vi "SMain.vi"() -> ()   [LabVIEW 2011] (continued)
                            n1009 = Build Path(base path=w1648, name or relative path="TXT\\ReportInf.txt" ("名称或相对路径")) -> (appended path=w1644:path)
                            n1010 = Write to Text File(file (use dialog)=w1644, text=w1645) -> ()  [unwired: 2 in, 3 out]
                          }
                          frame #14 {
                            # "生成报告"
                            n1011 = property on="MO:" class="Str"() -> ("Visible"=w1720:bool)  [unwired: 2 in, 2 out]
                            n1012 = case shown="真" w1720 {
                              tunnel: w1727 -> [_ w1752]
                              frame False {
                              }
                              frame True {
                                w1732 = "0"
                                w1733 = "1"
                                n1013 = property class="Str"(reference=w1752) -> (reference out=w1745:refnum<vi>, "Value"=w1746:string)  [unwired: 1 in, 1 out]
                                n1014 = local read "DB1"() -> (w1728:T8)
                                n1015 = local read "test result"() -> (w1743:bool)
                                n1016 = local read "MO:"() -> (w1750:string)
                                n1017 = local read "P/N:"() -> (w1751:string)
                                n1018 = call "按工单数量查询.vi"("MO"=w1750, "DBSet"=w1728, "test result"=w1743, "PN"=w1751) -> ("当前数量"=w1742:string)  [unwired: 5 in]
                                n1019 = Decimal String To Number(string=w1742) -> (number=w1741:i32)  [unwired: 2 in, 1 out]
                                n1020 = local write "Pro Num"(w1741) -> ()
                                n1021 = Concatenate Strings(w1746, "\n", "当前工单已生产：" ("字符串"), w1742, "条" ("字符串")) -> (w1744:string)
                                n1022 = local read "MO Num"() -> (w1739:i64)
                                n1023 = local read "Pro Num"() -> (w1740:i64)
                                n1024 = property class="Str"(reference=w1745, "Value"=w1744) -> ()  [unwired: 1 in, 2 out]
                                n1025 = Subtract(x=w1740, y=w1739) -> (x-y=w1737:i64)
                                n1026 = Greater?(x=w1737, y=i64 0) -> (0:w1735:bool)
                                n1027 = Greater?(x=w1737, y=i64 20) -> (0:w1734:bool)
                                n1028 = Select(t=w1733, s=w1735, f=w1732) -> (s? t:f=w1731:string)
                                n1029 = Select(t=w1733, s=w1734, f=w1732) -> (s? t:f=w1730:string)
                                n1030 = Concatenate Strings(w1731, w1730) -> (w1729:string)
                                n1031 = case shown="\"10\"" w1729 {
                                frame "00", Default {
                                w1753 = u32 0
                                n1032 = property on="Pro Num" class="DigNum (严格)"("NumText.TextColor"=w1753) -> ()  [unwired: 2 in, 2 out]
                                n1033 = property on="P/N:" class="Str"("Text.TextColor"=w1753) -> ()  [unwired: 2 in, 2 out]
                                }
                                frame "10" {
                                w1754 = u32 16772608
                                n1034 = property on="Pro Num" class="DigNum (严格)"("NumText.TextColor"=w1754) -> ()  [unwired: 2 in, 2 out]
                                n1035 = property on="P/N:" class="Str"("Text.TextColor"=w1754) -> ()  [unwired: 2 in, 2 out]
                                }
                                frame "11" {
                                w1755 = u32 14423296
                                n1036 = property on="Pro Num" class="DigNum (严格)"("NumText.TextColor"=w1755) -> ()  [unwired: 2 in, 2 out]
                                n1037 = property on="P/N:" class="Str"("Text.TextColor"=w1755) -> ()  [unwired: 2 in, 2 out]
                                }
                                }
                              }
                            }
                            n1038 = local read "Report Temp. Name"() -> (w1725:string)
                            n1039 = local read "TXT Data Path"() -> (w1719:path)
                            n1040 = local read "Report Config"() -> (w1724:string[])
                            n1041 = local read "Report Inf"() -> (w1723:string[])
                            n1042 = local read "Excel?"() -> (w1726:bool)
                            n1043 = Strip Path(path=w1719) -> (stripped path=w1718:path)  [unwired: 1 out]
                            n1044 = case shown="真" w1726 {
                              tunnel: w1719 -> [_ w1757]
                              tunnel: w1725 -> [_ w1768]
                              tunnel: w1724 -> [_ w1769]
                              tunnel: w1723 -> [_ w1764]
                              tunnel: w1722 -> [_ w1758]
                              tunnel: w1718 -> [_ w1756]
                              frame False {
                              }
                              frame True {
                                n1045 = Index Array(array=w1769, index #1=0 ("索引")) -> (element #1=w1765:string, element #2=w1763:string)  [unwired: 1 in]
                                n1046 = String To Path(string=w1768) -> (path=w1767:path)
                                n1047 = call "Excel Config.vi"("Config String"=w1765) -> ("Start(0,0)"=w1772:cluster{i32, i32}[], "Sheet Number List"=w1771:i32[], "File Name List"=w1770:string[])  [unwired: 8 in]
                                n1048 = call "Excel Config.vi"("Config String"=w1763) -> ("Start(0,0)"=w1762:cluster{i32, i32}[])  [unwired: 8 in, 2 out]
                                n1049 = call "Excel Export.vi"("template Path"=w1767, "Data Basic Path"=w1757, "File Name List"=w1770, "Sheet Index List"=w1771, "Report Inf"=w1764, "Inf start"=w1762, "Sheet start(0,0)"=w1772, "Demo"=w1758, "Report Type"="Report Type:", "reportSavePath"=w1756, "StartPage"="Start Page", "EndPage"="End Page") -> ()  [unwired: 15 in, 1 out]
                              }
                            }
                            n1050 = local write "proBar"(u8 90 ("proBar")) -> ()
                          }
                          frame #15 {
                            (unwired) FALSE
                            # "上传测试数据"
                            n1051 = local read "EEPROMTF"() -> (w1777:bool)
                            n1052 = local read "upload"() -> (w1776:bool)
                            n1053 = local read "测试模式"() -> (w1775:bool)
                            n1054 = Or(x=w1776, y=w1777) -> (x .or. y?=w1774:bool)
                            n1055 = And(x=w1774, y=w1775) -> (x .and. y?=w1773:bool)
                            n1056 = case shown="真" w1773 {
                              tunnel: w1778 -> [_ w1780]
                              frame False {
                                n1057 = local write "proBar"(u8 99 ("proBar")) -> ()
                              }
                              frame True {
                                n1058 = case shown="假" w1780 {
                                frame True {
                                n1059 = local read "strFSN 原始SN"() -> (w1785:string)
                                n1060 = local read "NetPathCompress1"() -> (w1783:path)
                                n1061 = local read "NetCmdCompress"() -> (w1784:string)
                                n1062 = local read "NetPathCompress2"() -> (w1782:path)
                                n1063 = call <vilib>:"Application Directory.vi"() -> ("Application Directory"=w1788:path)
                                n1064 = Build Path(base path=w1788, name or relative path="Demo_data") -> (appended path=w1786:path)
                                n1065 = local read "EEPROMTF"() -> (w1793:bool)
                                n1066 = local read "db_VNA"() -> (w1791:string)
                                n1067 = local read "条码输出"() -> (w1789:string)
                                n1068 = local read "Excel?"() -> (w1792:bool)
                                n1069 = local read "P/N:"() -> (w1794:string)
                                n1070 = local read "S/N:"() -> (w1790:string)
                                n1071 = call "compressFiles-Demo.vi"("mis原始sn字符串"=w1785, "P/N:"=w1794, "NetPathCompress1"=w1783, "NetPathCompress2"=w1782, "NetCmdCompress"=w1784, "original Path"=w1786, "EEPROMTF"=w1793, "Excel?"=w1792, "db_VNA"=w1791, "S/N:"=w1790, "条码输出"=w1789) -> ()  [unwired: 5 in]
                                }
                                frame False {
                                n1072 = local read "重测原因"() -> (w1797:string)
                                n1073 = property on="测试模式" class="Ring (严格)"() -> ("RingText.Text"=w1796:string)  [unwired: 2 in, 2 out]
                                n1074 = property on="线别" class="Ring (严格)"() -> ("RingText.Text"=w1795:string)  [unwired: 2 in, 2 out]
                                n1075 = local read "MO:"() -> (w1798:string)
                                n1076 = local read "Current Testing Label/当前测试条码"() -> (w1809:string)
                                n1077 = local read "要烧录的时间和Sn"() -> (w1802:string)
                                n1078 = local read "NetCmdCompress"() -> (w1799:string)
                                n1079 = local read "NetPathCompress1"() -> (w1800:path)
                                n1080 = local read "customer date"() -> (w1808:string)
                                n1081 = local read "strFSN 原始SN"() -> (w1811:string)
                                n1082 = local read "NetPathCompress2"() -> (w1801:path)
                                n1083 = local read "未经进制转换的sn(客户 jin zhi sn)"() -> (w1803:string)
                                n1084 = local read "Shi jin zhi sn"() -> (w1807:string)
                                n1085 = local read "midVar_time_date"() -> (w1806:timestamp)
                                n1086 = Format Date/Time String(time format string (%c)="%Y%m%d" ("时间格式字符串(%c)"), seconds (now)=w1806) -> (date/time string=w1804:string)  [unwired: 1 in]
                                n1087 = local read "original Path"() -> (w1812:path)
                                n1088 = local read "EEPROMTF"() -> (w1817:bool)
                                n1089 = local read "db_VNA"() -> (w1815:string)
                                n1090 = local read "条码输出"() -> (w1813:string)
                                n1091 = local read "Excel?"() -> (w1816:bool)
                                n1092 = local read "P/N:"() -> (w1818:string)
                                n1093 = local read "S/N:"() -> (w1814:string)
                                n1094 = local read "要烧录的DateCode"() -> (w1810:string)
                                n1095 = call "compressFiles.vi"("original Path"=w1812, "重测原因"=w1797, "NetPathCompress2"=w1801, "EEPROMTF"=w1817, "Excel?"=w1816, "测试模式"=w1796, "db_VNA"=w1815, "P/N:"=w1818, "S/N:"=w1814, "测试线别"=w1795, "NetPathCompress1"=w1800, "NetCmdCompress"=w1799, "mis原始sn字符串"=w1811, "条码输出"=w1813, "eprm_datecode"=w1810, "eprm_dateAndsn"=w1802, "itsn_really"=w1809, "label_date"=w1808, "decimel_sn"=w1807, "label_sn"=w1803, "decimel_date"=w1804, "MO"=w1798) -> ()  [unwired: 6 in]
                                }
                                }
                                n1096 = local write "proBar"(u8 95 ("proBar")) -> ()
                              }
                            }
                          }
                          frame #16 {
                            n1097 = flat-sequence {
                              frame #0 {
                                n1098 = local read "AutoSN"() -> (w1819:bool)
                                n1099 = call "运行批处理.vi"() -> ()  [unwired: 12 in]
                                n1100 = local write "proBar"(u8 100 ("proBar")) -> ()
                                n1101 = case shown="假" w1819 {
                                frame False {
                                n1102 = local write "S/N:"("" ("S/N:")) -> ()
                                n1103 = property on="S/N:" class="Str"("DisabledEnum"=T17."Enabled" ("禁用")) -> ()  [unwired: 2 in, 2 out]
                                }
                                frame True {
                                n1104 = local write "S/N:"("automatic sn" ("S/N:")) -> ()
                                n1105 = property on="S/N:" class="Str"("DisabledEnum"=T17."Disabled and Grayed Out" ("禁用")) -> ()  [unwired: 2 in, 2 out]
                                }
                                }
                                n1106 = disable-structure shown="启用" {
                                frame Disabled {
                                n1107 = call <vilib>:"System Exec.vi"("run minimized? (F)"=TRUE, "command line"="taskkill /IM bartend.exe /F") -> ()  [unwired: 6 in, 4 out]
                                }
                                frame Enabled {
                                }
                                }
                              }
                              frame #1 {
                                w1827 = FALSE ("Urgent Stop")
                                w1831 = 0
                                n1108 = property on="Start Test" class="Bool"("DisabledEnum"=w1831) -> ()  [unwired: 2 in, 2 out]
                                n1109 = property on="Tab_Graph" class="TabCtl (严格)"("Value"=w1831) -> ()  [unwired: 2 in, 2 out]
                                n1110 = property on="Urgent Stop" class="Bool (严格)"("DisabledEnum"=2 ("索引")) -> ()  [unwired: 2 in, 2 out]
                                n1111 = local write "State"("wait" ("state")) -> ()
                                n1112 = local write "Urgent Stop"(w1827) -> ()
                                n1113 = global write "全局.vi" "manual stop"(w1827) -> ()
                                n1114 = property on="S/N:" class="Str"("Key Focus"=TRUE ("键选中")) -> ()  [unwired: 2 in, 2 out]
                              }
                            }
                          }
                        }
                      }
                    }
                  }
                }
              }
              frame #3 {
                n1115 = local read "caliFlag"() -> (w1832:string)
                n1116 = case shown="\"假\", 默认" w1832 {
                  frame "假", Default {
                  }
                  frame "cali" {
                    n1117 = local write "State"("datacheck" ("state")) -> ()
                    n1118 = property on="Start Test" class="Bool"("DisabledEnum"=T17."Disabled and Grayed Out" ("禁用")) -> ()  [unwired: 2 in, 2 out]
                    n1119 = property on="Tab_Graph" class="TabCtl (严格)"("Value"=T15."Sxxxx1" ("Tab_Graph")) -> ()  [unwired: 2 in, 2 out]
                  }
                }
              }
            }
          }
          frame "datacheck" {
            n1120 = stacked-sequence {
              frame #0 {
                n1121 = local read "original Path"() -> (w1841:path)
                n1122 = Build Path(base path=w1841, name or relative path="txt" ("名称或相对路径")) -> (appended path=w1836:path)
                n1123 = call "caliCalcu.vi"("basic"=w1836) -> ("FileExsit"=w1839:bool, "keyValue"=w1838:string[][])  [unwired: 9 in]
                n1124 = case shown="真" w1839 {
                  tunnel: w1838 -> [_ w1850]
                  tunnel: [_ w1851] -> w1837
                  frame False {
                  }
                  frame True {
                    n1125 = local read "sampleData"() -> (w1857:string)
                    n1126 = Spreadsheet String To Array(format string="%f" ("格式字符串"), spreadsheet string=w1857, array type (2D Dbl)=dbl[][] []) -> (array=w1856:dbl[][])  [unwired: 1 in]
                    n1127 = Fract/Exp String To Number(string=w1850) -> (number=w1854:dbl[][])  [unwired: 3 in, 1 out]
                    n1128 = Subtract(x=w1854, y=w1856) -> (x-y=w1847:dbl[][])
                    n1129 = Array To Spreadsheet String(array=w1850, 3:"%f" ("格式字符串")) -> (spreadsheet string=→"caliData":string)  [unwired: 1 in]
                    n1130 = Absolute Value(x=w1854) -> (abs(x)=w1845:dbl[][])
                    n1131 = Absolute Value(x=w1847) -> (abs(x)=w1846:dbl[][])
                    n1132 = Divide(x=w1846, y=w1845) -> (x/y=w1853:dbl[][])
                    n1133 = Less Or Equal?(x=w1853, y=0.1) -> (x <= y?=w1843:bool[][])
                    n1134 = Not A Number/Path/Refnum?(number/path/refnum=w1845) -> (NaN/Path/Refnum?=w1844:bool[][])
                    n1135 = Or(x=w1844, y=w1843) -> (x .or. y?=w1842:bool[][])
                    n1136 = And Array Elements(Boolean array=w1842) -> (logical AND=w1851:bool)
                  }
                }
                "caliPassed" <- w1837
              }
              frame #1 {
                n1137 = local read "caliPassed"() -> (w1859:bool)
                n1138 = case shown="假" w1859 {
                  frame False {
                    n1139 = One Button Dialog(message="校准数据超出10%范围，未通过" ("消息")) -> ()  [unwired: 1 in, 1 out]
                  }
                  frame True {
                    n1140 = local read "caliData"() -> (w1861:string)
                    n1141 = local read "SystemMode"() -> (w1866:string)
                    n1142 = Format Date/Time String() -> (date/time string=w1865:string)  [unwired: 3 in]
                    n1143 = property on="sampleNo" class="Ring (严格)"() -> ("RingText.Text"=w1870:string)  [unwired: 2 in, 2 out]
                    n1144 = property on="Type" class="Ring (严格)"() -> ("RingText.Text"=w1869:string)  [unwired: 2 in, 2 out]
                    n1145 = Build Array(w1870, w1869, "Figo", "PASS", w1866, w1861, w1865) -> (w1864:string[])
                    n1146 = for {
                      shift-right: [w1875] -> w1863
                      shift-left: "INSERT INTO dbo.cali_log (goldenSampleNo, type, caliUser, result, setNo, detail, caliDate)\nVALUES ('@goldensampleno', '@type', '@caliuser', '@result', '@setno', '@detail', '@calidate')" -> [w1876]
                      tunnel: string[] ["@goldensampleno", "@type", "@caliuser", "@result", "@setno", "@detail", "@calidate"] -> [w1874] mode=indexing
                      tunnel: w1864 -> [w1873] mode=indexing
                      n1147 = Search and Replace String(input string=w1876, search string=w1874, replace string=w1873) -> (result string=w1875:string)  [unwired: 5 in, 3 out]
                    }
                    n1148 = local read "DB1"() -> (w1862:T8)
                    n1149 = call "query.net.vi"("Sql"=w1863, "DBSet"=w1862) -> ()  [unwired: 8 in, 2 out]
                  }
                }
              }
              frame #2 {
                n1150 = local read "caliPassed"() -> (w1877:bool)
                n1151 = case shown="真" w1877 {
                  frame False {
                  }
                  frame True {
                    n1152 = One Button Dialog(message="校准通过，可以开始测试" ("消息")) -> ()  [unwired: 1 in, 1 out]
                  }
                }
              }
              frame #3 {
                n1153 = local write "State"("wait" ("State")) -> ()
              }
              frame #4 {
                n1154 = local read "P/N:"() -> (w1880:string)
                n1155 = property on="P/N:" class="Str"("Val(Sgnl)"=w1880) -> ()  [unwired: 2 in, 2 out]
              }
            }
          }
          frame "exit" {
          }
          frame "wait", Default {
            n1156 = event shown="[12] 菜单选择(用户)" {
              selector: _ -> [_ _ _ _ _ _ _ _ _ _ _ _ _ _ _ _ _ _ _ _]
              dyn-events: _ -> [_ _ _ _ _ _ _ _ _ _ _ _ _ _ _ _ _ _ _ _]
              timeout: _ -> [_ _ _ _ _ _ _ _ _ _ _ _ _ _ _ _ _ _ _ _]
              tunnel: ["Stop" _ _ w1934 _ _ _ _ _ _ _ _ _ _ _ _ _ _ _ _] -> w1882
              event "Stop": Value Change {
                n1157 = event-data() -> ()  [unwired: 1 in, 5 out]
              }
              event "save config": Value Change {
                n1158 = event-data() -> ()  [unwired: 1 in, 5 out]
                n1159 = case shown="真" "save config" {
                  frame False {
                  }
                  frame True {
                    n1160 = stacked-sequence {
                      seq-local: [w1891 _ _] -> [_ w1922 _]
                      frame #0 {
                        n1161 = local read "Crosstalk  by Trace"() -> (w1902:bool)
                        n1162 = local read "Local Database"() -> (w1905:bool)
                        n1163 = local read "By Channel?"() -> (w1890:bool)
                        n1164 = local read "Use Counts?"() -> (w1887:bool)
                        n1165 = property on="VNA Model:" class="Enum (严格)"() -> ("RingText.Text"=w1909:string)  [unwired: 2 in, 2 out]
                        n1166 = property on="DAQ  Model:" class="Enum (严格)"() -> ("RingText.Text"=w1908:string)  [unwired: 2 in, 2 out]
                        n1167 = property on="DAQ Device" class="Ring (严格)"() -> ("RingText.Text"=w1907:string)  [unwired: 2 in, 2 out]
                        n1168 = local read "Dem 2X"() -> (w1901:bool)
                        n1169 = local read "Manual"() -> (w1903:bool)
                        n1170 = property on="VNA VISA" class="VISAName"() -> ("Text.Text"=w1910:string)  [unwired: 2 in, 2 out]
                        n1171 = property on="VISA COM" class="VISAName"() -> ("Text.Text"=w1906:string)  [unwired: 2 in, 2 out]
                        n1172 = local read "Demo"() -> (w1904:bool)
                        n1173 = property on="RS232 I2C Counts" class="VISAName"() -> ("Text.Text"=w1885:string)  [unwired: 2 in, 2 out]
                        n1174 = Build Array(FALSE ("元素"), w1905, w1904, w1903, w1902, w1901, w1890) -> (w1900:bool[])
                        n1175 = property on="打印模式" class="Enum (严格)"() -> ("RingText.Text"=w1893:string)  [unwired: 2 in, 2 out]
                        n1176 = property on="Adaptor:" class="Enum (严格)"() -> ("RingText.Text"=w1892:string)  [unwired: 2 in, 2 out]
                        n1177 = for {
                          tunnel: w1900 -> [w1921] mode=indexing
                          tunnel: [w1918] -> w1898 mode=indexing
                          n1178 = Select(t="TRUE", s=w1921, f="FALSE") -> (s? t:f=w1918:string)
                        }
                        n1179 = local read "upload"() -> (w1914:bool)
                        n1180 = property on="Printer VISA" class="VISAName"() -> ("Text.Text"=w1896:string)  [unwired: 2 in, 2 out]
                        n1181 = property on="RS232 I2C VISA" class="VISAName"() -> ("Text.Text"=w1911:string)  [unwired: 2 in, 2 out]
                        n1182 = Build Array(w1910, w1909, w1908, w1907, w1906) -> (w1899:string[])
                        n1183 = Insert Into Array(array=w1899, new element=w1898) -> (w1897:string[])  [unwired: 1 in]
                        n1184 = Select(t="TRUE", s=w1914, f="FALSE") -> (s? t:f=w1915:string)
                        n1185 = local read "Port Type"() -> (w1916:u16)
                        n1186 = Select(t="TRUE", s=w1887, f="FALSE") -> (s? t:f=w1886:string)
                        n1187 = Number To Decimal String(number=w1916) -> (decimal integer string=w1917:string)  [unwired: 1 in]
                        n1188 = Build Array(w1896, w1911, w1915, w1917, w1893, w1892, w1886, w1885) -> (w1895:string[])
                        n1189 = Insert Into Array(array=w1897, new element=w1895) -> (w1891:string[])  [unwired: 1 in]
                      }
                      frame #1 {
                        n1190 = call <vilib>:"Application Directory.vi"() -> ("Application Directory"=w1927:path)
                        n1191 = Build Path(base path=w1927, name or relative path="database\\initializeConfig.txt" ("名称或相对路径")) -> (appended path=w1924:path)
                        n1192 = call-poly <vilib>:"Read From Spreadsheet File.vi"("file path (dialog if empty)"=w1924) -> ("all rows"=w1926:string[][])  [unwired: 6 in, 4 out]
                        n1193 = Replace Array Subset(array=w1926, new element=w1922, index (col)=1 ("禁用的索引 (列)")) -> (w1923:string[][])  [unwired: 1 in]
                        n1194 = call-poly <vilib>:"Write To Spreadsheet File.vi"("2D data"=w1923, "file path (dialog if empty)"=w1924) -> ()  [unwired: 6 in, 1 out]
                      }
                      frame #2 {
                        n1195 = Wait (ms)(milliseconds to wait=u32 200 ("等待时间（毫秒）")) -> ()  [unwired: 1 out]
                      }
                    }
                  }
                }
              }
              event "打印模式": Value Change {
                n1196 = event-data() -> ("NewVal"=w1930:enum16{"IT Print", "EE Print"})  [unwired: 1 in, 4 out]
                n1197 = case shown="\"IT Print\", 默认" w1930 {
                  frame "IT Print", Default {
                    n1198 = property on="MO:" class="Str"("Visible"=TRUE ("可见")) -> ()  [unwired: 2 in, 2 out]
                    n1199 = local write "EE Write"(TRUE ("EE Write")) -> ()
                  }
                  frame "EE Print" {
                    n1200 = property on="MO:" class="Str"("Visible"=FALSE ("可见")) -> ()  [unwired: 2 in, 2 out]
                  }
                }
              }
              event Panel Close {
                n1201 = event-data() -> ()  [unwired: 1 in, 3 out]
                n1202 = flat-sequence {
                  tunnel: [FALSE ("Stop")] -> w1934
                  frame #0 {
                  }
                  frame #1 {
                  }
                  frame #2 {
                    n1203 = local write "State"("exit" ("state")) -> ()
                  }
                }
              }
              event "Report Type:": Value Change {
                n1204 = event-data() -> ("NewVal"=w1939:u16)  [unwired: 1 in, 4 out]
                n1205 = case shown="1" w1939 {
                  tunnel: [w1940 w1941] -> w1938
                  tunnel: [w1940 w1941] -> w1937
                  frame 0, Default {
                    w1940 = FALSE ("可见")
                  }
                  frame 1 {
                    w1941 = TRUE ("可见")
                  }
                }
                n1206 = property on="Start Page" class="DigNum (严格)"("Visible"=w1938) -> ()  [unwired: 2 in, 2 out]
                n1207 = property on="End Page" class="DigNum (严格)"("Visible"=w1937) -> ()  [unwired: 2 in, 2 out]
              }
              event "VNA VISA": Value Change {
                n1208 = event-data() -> ()  [unwired: 1 in, 5 out]
                n1209 = property on="VNA VISA" class="VISAName"() -> ("Text.Text"=w1942:string)  [unwired: 2 in, 2 out]
                n1210 = Search/Split String(string=w1942, search string/char (-)="N5224A" ("搜索字符串/字符(-)")) -> (offset of match=w1945:i32)  [unwired: 1 in, 2 out]
                n1211 = case shown="-1" w1945 {
                  tunnel: [w1951 0] -> w1944
                  tunnel: [w1950 2] -> w1943
                  tunnel: w1942 -> [w1948 _]
                  frame -1 {
                    n1212 = Search/Split String(string=w1948, search string/char (-)="E5071C" ("搜索字符串/字符(-)")) -> (offset of match=w1947:i32)  [unwired: 1 in, 2 out]
                    n1213 = case shown="-1" w1947 {
                      tunnel: [1 1] -> w1951
                      tunnel: [0 1] -> w1950
                      frame 0..20, Default {
                      }
                      frame -1 {
                      }
                    }
                  }
                  frame 1..20, Default {
                  }
                }
                n1214 = property on="VNA Model:" class="Enum (严格)"("Value"=w1943) -> ()  [unwired: 2 in, 2 out]
                n1215 = property on="Port Type" class="Ring (严格)"("Value"=w1944) -> ()  [unwired: 2 in, 2 out]
              }
              event "VNA Model:": Value Change {
                n1216 = event-data() -> ()  [unwired: 1 in, 5 out]
                n1217 = case shown="\"N5224A\"" "VNA Model:" {
                  tunnel: [u16 1 ("Port Type") u16 1 ("Port Type") u16 0 ("Port Type")] -> w1958
                  frame "E5071C", Default {
                  }
                  frame "N5230A(C)" {
                  }
                  frame "N5224A" {
                  }
                }
                n1218 = property on="Port Type" class="Ring (严格)"("Value"=w1958) -> ()  [unwired: 2 in, 2 out]
              }
              event "Urgent Stop": Value Change {
                n1219 = event-data() -> ("NewVal"=w1963:bool)  [unwired: 1 in, 4 out]
                n1220 = local write "Urgent Stop"(w1963) -> ()
                n1221 = global write "全局.vi" "manual stop"(w1963) -> ()
              }
              event "Manual": Value Change {
                n1222 = event-data() -> ()  [unwired: 1 in, 5 out]
                n1223 = local read "Manual"() -> (w1965:bool)
                n1224 = local read "Demo"() -> (w1964:bool)
                n1225 = local read "DAQ  Model:"() -> (w1968:T14)
                n1226 = local read "DAQ Device"() -> (w1967:u16)
                n1227 = local read "VISA COM"() -> (w1969:refnum<visa-resource-name>)
                n1228 = Or(x=w1965, y=w1964) -> (x .or. y?=w1966:bool)
                n1229 = case shown="假" w1966 {
                  tunnel: w1967 -> [w1972 _]
                  tunnel: w1968 -> [w1971 _]
                  tunnel: w1969 -> [w1970 _]
                  frame False {
                    n1230 = case shown="\"LX MCU\"" w1971 {
                      tunnel: w1972 -> [w1977 _ _]
                      tunnel: w1970 -> [_ w1979 w1981]
                      frame "NI PCI-6509", Default {
                        n1231 = local read "Switch array"() -> (w1975:bool[][])
                        n1232 = call "6509 simple.vi"("error in"="error in 2", "index (row)"=i8 39, "array input: P0-P1-P2-P3-P4-P5"=w1975, "DAQ device"=w1977) -> ("error out"=→"error out 2":errorcluster)  [unwired: 3 in]
                      }
                      frame "LX MCU" {
                        w1978 = u16 1 items=["Testing", "Close All"] ("Function")
                        n1233 = call "MCU Switch Control.vi"("Function"=w1978, "VISA"=w1979) -> ()  [unwired: 9 in, 1 out]
                      }
                      frame "LX MCU_40G" {
                        w1980 = u16 1 items=["Testing", "Close All"] ("Function")
                        n1234 = call "40G MCU Switch Control.vi"("Function"=w1980, "VISA"=w1981) -> ()  [unwired: 9 in, 1 out]
                      }
                    }
                  }
                  frame True {
                  }
                }
              }
              event "DAQ  Model:": Value Change {
                n1235 = event-data() -> ()  [unwired: 1 in, 5 out]
                n1236 = local read "DAQ  Model:"() -> (w1984:T14)
                n1237 = case shown="\"LX MCU_40G\"" w1984 {
                  tunnel: [2 0 0] -> w1983
                  tunnel: [0 2 2] -> w1982
                  frame "NI PCI-6509", Default {
                  }
                  frame "LX MCU" {
                  }
                  frame "LX MCU_40G" {
                  }
                }
                n1238 = property on="DAQ Device" class="Ring (严格)"("DisabledEnum"=w1982) -> ()  [unwired: 2 in, 2 out]
                n1239 = property on="VISA COM" class="VISAName"("DisabledEnum"=w1983) -> ()  [unwired: 2 in, 2 out]
              }
              event Key Down {
                n1240 = event-data() -> ("ScanCode"=w1993:i16)  [unwired: 1 in, 8 out]
                n1241 = disable-structure shown="启用" {
                  frame Disabled {
                    n1242 = call "keyboard_VNA_jet.vi"() -> ()  [unwired: 9 in, 1 out]
                  }
                  frame Enabled {
                  }
                }
                n1243 = local read "midVar_bool_find"() -> (w1995:bool)
                n1244 = Equal?(x=w1993, y=i16 28) -> (x = y?=w1991:bool)
                n1245 = And(x=w1991, y=w1995) -> (x .and. y?=w1994:bool)
                n1246 = case shown="真" w1994 {
                  frame False {
                    n1247 = local write "State"("wait" ("state")) -> ()
                  }
                  frame True {
                    n1248 = flat-sequence {
                      frame #0 {
                        n1249 = property on="P/N:" class="Str"("Key Focus"=FALSE ("键选中")) -> ()  [unwired: 2 in, 2 out]
                      }
                      frame #1 {
                        n1250 = local read "S/N:"() -> (w1999:string)
                        n1251 = Empty String/Path?(string/path=w1999) -> (empty?=w1998:bool)
                        n1252 = case shown="假" w1998 {
                          frame False {
                            n1253 = local write "State"("test" ("state")) -> ()
                          }
                          frame True {
                            n1254 = local write "State"("wait" ("state")) -> ()
                            n1255 = One Button Dialog(message="SN不能为空！") -> ()  [unwired: 1 in, 1 out]
                          }
                        }
                      }
                    }
                  }
                }
              }
              event "Start Test": Value Change {
                n1256 = event-data() -> ()  [unwired: 1 in, 5 out]
                n1257 = local read "midVar_bool_find"() -> (w2003:bool)
                n1258 = case shown="真" w2003 {
                  frame False {
                    n1259 = local write "State"("wait" ("state")) -> ()
                  }
                  frame True {
                    n1260 = local read "S/N:"() -> (w2006:string)
                    n1261 = Empty String/Path?(string/path=w2006) -> (empty?=w2005:bool)
                    n1262 = case shown="假" w2005 {
                      frame False {
                        (unwired) "datacheck" ("State")
                        n1263 = local write "State"("test" ("state")) -> ()
                      }
                      frame True {
                        n1264 = local write "State"("wait" ("state")) -> ()
                        n1265 = One Button Dialog(message="SN不能为空！") -> ()  [unwired: 1 in, 1 out]
                      }
                    }
                  }
                }
              }
              event Menu Selection (User) {
                n1266 = event-data() -> ("MenuRef"=w2013:refnum<k9>, "ItemTag"=w2014:string)  [unwired: 1 in, 4 out]
                n1267 = control-ref of="Test Status:"() -> (w2011:refnum<vi>)
                n1268 = local read "DB1"() -> (w2010:T8)
                n1269 = case shown="\"Project Management\"" w2014 {
                  selector: w2014 -> [_ _ _ _ _ _ _ _ _ _ _ _ w2056 w2069 _]
                  tunnel: w2013 -> [_ _ _ _ _ _ _ _ _ _ _ _ w2055 w2068 _]
                  tunnel: "error in" -> [w2015 _ _ _ _ _ _ _ _ _ _ _ _ _ _]
                  tunnel: w2011 -> [_ _ _ _ _ _ _ _ w2037 _ _ _ _ _ _]
                  tunnel: w2010 -> [_ _ _ w2019 w2028 _ _ _ _ _ _ _ w2052 w2065 _]
                  frame "6509 Switch Tool", Default {
                    n1270 = call "RF Switch tool.vi"("error in"=w2015) -> ("Error out"=→"error out":errorcluster)  [unwired: 6 in]
                  }
                  frame "MCU Switch Tool" {
                    n1271 = local read "DAQ  Model:"() -> (w2017:T14)
                    n1272 = case shown="\"LX MCU_40G_HuaWei\"" w2017 {
                      frame "LX MCU", Default {
                        n1273 = call "RF Switch tool by MCU.vi"() -> ()  [unwired: 8 in]
                      }
                      frame "LX MCU_40G_HuaWei" {
                        n1274 = call "RF Switch tool by MCU HuaWei.vi"() -> ()  [unwired: 8 in]
                      }
                      frame "LX MCU_40G" {
                        n1275 = call "40G RF Switch Matrix.vi"() -> ()  [unwired: 8 in]
                      }
                    }
                  }
                  frame "40G 6509" {
                    n1276 = call "40G RF Switch Tool(NI 6509).vi"() -> ()  [unwired: 8 in]
                  }
                  frame "Project Management" {
                    n1277 = call "LoginForm.vi"("DBSet"=w2019) -> ("登录成功"=w2023:bool, "用户名"=w2022:string, "loginMode"=w2018:bool, "厂区"=w2021:string)
                    n1278 = local read "DB2"() -> (w2020:T8)
                    n1279 = case shown="真" w2023 {
                      tunnel: w2022 -> [_ w2026]
                      tunnel: w2021 -> [_ w2027]
                      tunnel: w2020 -> [_ w2025]
                      tunnel: w2018 -> [_ _]
                      frame False {
                        n1280 = One Button Dialog(message="密码或用户名错误" ("消息")) -> ()  [unwired: 1 in, 1 out]
                      }
                      frame True {
                        n1281 = call "New Project.vi"("DBSet"=w2025, "UserID"=w2026, "厂区"=w2027) -> ()  [unwired: 9 in]
                      }
                    }
                  }
                  frame "SampleImport" {
                    n1282 = call "LoginForm.vi"("DBSet"=w2028) -> ("登录成功"=w2032:bool, "用户名"=w2031:string, "厂区"=w2030:string)  [unwired: 1 out]
                    n1283 = local read "DB2"() -> (w2029:T8)
                    n1284 = case shown="真" w2032 {
                      tunnel: w2031 -> [_ w2036]
                      tunnel: w2030 -> [_ _]
                      tunnel: w2029 -> [_ _]
                      tunnel: w2028 -> [_ w2035]
                      frame False {
                        n1285 = One Button Dialog(message="密码或用户名错误" ("消息")) -> ()  [unwired: 1 in, 1 out]
                      }
                      frame True {
                        n1286 = local read "SystemMode"() -> (w2034:string)
                        n1287 = call "importNewSample.vi"("DBSet"=w2035, "setNo"=w2034, "user"=w2036) -> ()  [unwired: 9 in]
                      }
                    }
                  }
                  frame "Fixture Management" {
                  }
                  frame "S4P Data Tool" {
                    n1288 = call "S4P Tool.vi"() -> ()  [unwired: 12 in]
                  }
                  frame "EEPROM Editor" {
                    n1289 = call "SubMain2_ChartEEPROM_vna_wmg.vi"() -> ()  [unwired: 12 in]
                  }
                  frame "Label Debug" {
                    n1290 = local read "打印模式"() -> (w2038:enum16{"IT Print", "EE Print"})
                    n1291 = case shown="\"IT Print\", 默认" w2038 {
                      tunnel: w2037 -> [w2046 _]
                      frame "IT Print", Default {
                        n1292 = local read "PRINT"() -> (w2048:refnum<k24>)
                        n1293 = local read "P/N:"() -> (w2047:string)
                        n1294 = local read "DB1"() -> (w2039:T8)
                        n1295 = local read "Fast Print"() -> (w2040:bool)
                        n1296 = local read "SN"() -> (w2049:refnum<k24>)
                        n1297 = property class="Str"(reference=w2046) -> (reference out=w2042:refnum<vi>, "Value"=w2045:string)  [unwired: 1 in, 1 out]
                        n1298 = call "资讯重打标签.vi"("DBSet"=w2039, "print path local"=w2040, "PN"=w2047, "PRINT"=w2048, "SN"=w2049) -> ("PrintMsg"=w2043:string)  [unwired: 6 in]
                        n1299 = Concatenate Strings(w2045, "\n", w2043) -> (w2041:string)
                        n1300 = property class="Str"(reference=w2042, "Value"=w2041) -> ()  [unwired: 1 in, 2 out]
                      }
                      frame "EE Print" {
                        n1301 = call "re-print.vi"() -> ()  [unwired: 12 in]
                      }
                    }
                  }
                  frame "Impedance Test Tool" {
                    n1302 = call "Impedance Testing Tool.vi"() -> ()  [unwired: 12 in]
                  }
                  frame "Control Counting module" {
                    n1303 = call "登录对话框.vi"() -> ("登录状态"=w2050:bool)  [unwired: 3 in, 3 out]
                    n1304 = case shown="真" w2050 {
                      frame False {
                      }
                      frame True {
                        n1305 = local read "RS232 I2C Counts"() -> (w2051:refnum<visa-resource-name>)
                        n1306 = call "初始化使用次数和寿命的界面.vi"("VISA  2"=w2051) -> ()  [unwired: 11 in]
                      }
                    }
                  }
                  frame "Eeprom Write Delay Config" {
                    n1307 = call "saveDelayConfig_烧录.vi"() -> ()  [unwired: 9 in, 3 out]
                  }
                  frame "Excel Data Export" {
                    n1308 = Get Menu Item Info(7:w2056, 11:w2055) -> (0:w2059:errorcluster, 2:w2058:string, 3:w2060:refnum<k9>, 4:w2057:bool)  [unwired: 1 in, 3 out]
                    n1309 = Not(x=w2057) -> (.not. x?=w2054:bool)
                    n1310 = case shown="假" w2054 {
                      selector: w2054 -> [_ w2064]
                      tunnel: [w2063 w2064] -> w2053
                      tunnel: w2052 -> [w2061 _]
                      frame False {
                        n1311 = call "LoginForm.vi"("DBSet"=w2061) -> ("登录成功"=w2062:bool)  [unwired: 3 out]
                        n1312 = Not(x=w2062) -> (.not. x?=w2063:bool)
                      }
                      frame True {
                      }
                    }
                    "Excel?" <- w2053
                    n1313 = Set Menu Item Info(6:w2053, 7:w2056, 8:w2059, 10:w2058, 11:w2060) -> ()  [unwired: 2 in, 2 out]
                  }
                  frame "Data UpLoad" {
                    n1314 = Get Menu Item Info(7:w2069, 11:w2068) -> (0:w2072:errorcluster, 2:w2071:string, 3:w2073:refnum<k9>, 4:w2070:bool)  [unwired: 1 in, 3 out]
                    n1315 = Not(x=w2070) -> (.not. x?=w2067:bool)
                    n1316 = case shown="假" w2067 {
                      selector: w2067 -> [_ w2077]
                      tunnel: [w2076 w2077] -> w2066
                      tunnel: w2065 -> [w2074 _]
                      frame False {
                        n1317 = call "LoginForm.vi"("DBSet"=w2074) -> ("登录成功"=w2075:bool)  [unwired: 3 out]
                        n1318 = Not(x=w2075) -> (.not. x?=w2076:bool)
                      }
                      frame True {
                      }
                    }
                    "upload" <- w2066
                    n1319 = Set Menu Item Info(6:w2066, 7:w2069, 8:w2072, 10:w2071, 11:w2073) -> ()  [unwired: 2 in, 2 out]
                  }
                  frame "Help" {
                    n1320 = call "Help.vi"() -> ()  [unwired: 20 in]
                  }
                }
              }
              event "Type": Value Change {
                n1321 = event-data() -> ()  [unwired: 1 in, 5 out]
                n1322 = local read "SystemMode"() -> (w2088:string)
                n1323 = property on="Type" class="Ring (严格)"() -> ("RingText.Text"=w2084:string)  [unwired: 2 in, 2 out]
                n1324 = Search and Replace String(input string="SELECT goldenSampleNo,caiData FROM cali_sample WHERE setNo='@SystemMode@' AND status='1' and type='@type@'", search string="@SystemMode@" ("搜索字符串"), replace string=w2088) -> (result string=w2086:string)  [unwired: 5 in, 3 out]
                n1325 = Search and Replace String(input string=w2086, search string="@type@" ("搜索字符串"), replace string=w2084) -> (result string=w2083:string)  [unwired: 5 in, 3 out]
                n1326 = local read "DB1"() -> (w2087:T8)
                n1327 = call "query.net.vi"("Sql"=w2083, "DBSet"=w2087) -> ("result"=w2082:string[][])  [unwired: 8 in, 1 out]
                n1328 = Index Array(array=w2082, index (col)=0 ("禁用的索引 (列)")) -> (element=w2080:string[])  [unwired: 1 in]
                n1329 = property on="sampleNo" class="Ring (严格)"("Strings []"=w2080) -> ()  [unwired: 2 in, 2 out]
                n1330 = Array Size(array=w2080) -> (size(s)=w2079:i32)
                n1331 = Greater Than 0?(x=w2079) -> (x > 0?=w2078:bool)
                n1332 = case shown="假" w2078 {
                  frame False {
                    n1333 = property on="sampleNo" class="Ring (严格)"("Val(Sgnl)"=u16 0 ("值(信号)")) -> ()  [unwired: 2 in, 2 out]
                  }
                  frame True {
                    n1334 = property on="sampleNo" class="Ring (严格)"("Val(Sgnl)"=u16 0 ("值(信号)")) -> ()  [unwired: 2 in, 2 out]
                  }
                }
              }
              event "sampleNo": Value Change {
                n1335 = event-data() -> ()  [unwired: 1 in, 5 out]
                n1336 = property on="sampleNo" class="Ring (严格)"() -> ("RingText.Text"=w2102:string)  [unwired: 2 in, 2 out]
                n1337 = Search and Replace String(input string="SELECT caiData FROM cali_sample WHERE goldenSampleNo='@goldenSampleNoe@' AND status='1'", search string="@goldenSampleNoe@" ("搜索字符串"), replace string=w2102) -> (result string=w2101:string)  [unwired: 5 in, 3 out]
                n1338 = local read "DB1"() -> (w2103:T8)
                n1339 = call "query.net.vi"("Sql"=w2101, "DBSet"=w2103) -> ("result"=w2100:string[][])  [unwired: 8 in, 1 out]
                n1340 = Index Array(array=w2100, index (row)=0 ("索引 (行)")) -> (element=w2095:string[])  [unwired: 1 in]
                n1341 = Array Size(array=w2095) -> (size(s)=w2098:i32)
                n1342 = Equal?(x=w2098, y=1) -> (x = y?=w2096:bool)
                n1343 = case shown="真" w2096 {
                  tunnel: w2095 -> [_ w2110]
                  tunnel: [_ w2108] -> w2094
                  tunnel: [FALSE TRUE] -> w2093
                  frame False {
                  }
                  frame True {
                    n1344 = Index Array(array=w2110, index=0 ("索引")) -> (element=w2108:string)
                  }
                }
                "sampleData" <- w2094
                "caliDataSelect" <- w2093
              }
              event "P/N:": Value Change {
                n1345 = event-data() -> ()  [unwired: 1 in, 5 out]
                n1346 = property on="线别" class="Ring (严格)"() -> ("RingText.Text"=w2116:string)  [unwired: 2 in, 2 out]
                n1347 = local read "SystemMode"() -> (w2118:string)
                n1348 = Concatenate Strings("当前线别为：" ("字符串"), w2116, "是否正确" ("字符串")) -> (w2114:string)
                n1349 = Two Button Dialog(message=w2114) -> (T button?=w2113:bool)  [unwired: 2 in]
                "线别确认" <- w2113
                n1350 = local read "DB2"() -> (w2111:T8)
                n1351 = property on="线别" class="Ring (严格)"("DisabledEnum"=T17."Enabled" ("禁用")) -> ()  [unwired: 2 in, 2 out]
                n1352 = case shown="假" w2113 {
                  frame False {
                  }
                  frame True {
                    n1353 = property on="线别" class="Ring (严格)"("DisabledEnum"=T17."Disabled and Grayed Out" ("禁用")) -> ()  [unwired: 2 in, 2 out]
                  }
                }
                n1354 = local write "AutoSN"(FALSE ("AutoSN")) -> ()
                n1355 = local read "Demo"() -> (w2121:bool)
                n1356 = call "Query Project by PN.vi"("Luxshare_P/N:"="P/N:", "System_Mode"=w2118, "Local"="Local Database", "DBSet"=w2111) -> ("Find?"=w2122:bool, "Basic Information"=w2127:string[], "Project  Information"=w2128:string[][], "limitSpec"=w2126:string[][], "SwitchMatrix"=w2125:i32[][], "Label Content"=w2124:string)  [unwired: 9 in, 1 out]
                n1357 = case shown="真" w2122 {
                  tunnel: w2128 -> [_ w2140]
                  tunnel: w2127 -> [_ w2139]
                  tunnel: w2126 -> [_ w2137]
                  tunnel: w2125 -> [_ w2138]
                  tunnel: w2124 -> [_ w2135]
                  tunnel: w2121 -> [_ w2136]
                  tunnel: "P/N:" -> [_ w2134]
                  frame False {
                    w2131 = 2 ("索引")
                    w2132 = "" ("P/N:")
                    n1358 = local write "Sample Description"(w2132) -> ()
                    n1359 = local write "P/N:"(w2132) -> ()
                    n1360 = property on="Start Test" class="Bool"("DisabledEnum"=w2131) -> ()  [unwired: 2 in, 2 out]
                    n1361 = property on="VNA Initial" class="Bool"("DisabledEnum"=w2131) -> ()  [unwired: 2 in, 2 out]
                    n1362 = local write "midVar_bool_find"(FALSE ("midVar_bool_find")) -> ()
                  }
                  frame True {
                    n1363 = global write "全局.vi" "print templete"(TRUE ("print templete")) -> ()
                    n1364 = stacked-sequence {
                      tunnel: w2140 -> [_ _ _ _ _ w2302 _ _ _ _ _ _ _ _ _]
                      tunnel: w2139 -> [_ w2191 w2228 w2234 w2237 _ _ _ _ _ _ _ w2475 _ _]
                      tunnel: w2138 -> [_ _ _ _ _ _ _ _ w2361 _ _ _ _ _ _]
                      tunnel: w2137 -> [_ _ _ _ w2235 w2279 _ _ _ _ _ _ _ _ _]
                      tunnel: w2136 -> [_ _ _ _ _ _ _ _ _ _ w2384 _ _ _ _]
                      tunnel: w2135 -> [_ w2175 _ _ _ _ _ _ _ _ _ _ _ _ _]
                      tunnel: w2134 -> [_ _ _ _ _ _ _ _ _ _ _ w2399 w2469 _ _]
                      frame #0 {
                        n1365 = local read "打印模式"() -> (w2143:enum16{"IT Print", "EE Print"})
                        n1366 = local write "MO Num"(i64 0 ("MO Num")) -> ()
                        n1367 = local write "Pro Num"(i64 0 ("Pro Num")) -> ()
                        n1368 = case shown="\"IT Print\", 默认" w2143 {
                          frame "IT Print", Default {
                            n1369 = local read "MO:"() -> (w2145:string)
                            n1370 = local read "P/N:"() -> (w2149:string)
                            n1371 = local read "SN"() -> (w2146:refnum<k24>)
                            n1372 = local write "EE Write"(TRUE ("EE Write")) -> ()
                            n1373 = call "资讯打标签-检测工单料号匹配.vi"("工单号"=w2145, "料号"=w2149, "引用"=w2146) -> ("工单号、料号检测情况"=w2148:string, "工单数量"=w2147:string)  [unwired: 9 in, 2 out]
                            n1374 = case shown="\"00\", 默认" w2148 {
                              tunnel: w2147 -> [_ _ w2160]
                              tunnel: w2145 -> [_ _ w2159]
                              frame "00", Default {
                                n1375 = local write "midVar_bool_find"(FALSE ("midVar_bool_find")) -> ()
                                n1376 = One Button Dialog(message="工单不存在,输入错误或者线长没有在Tiptop中激活！" ("消息")) -> ()  [unwired: 1 in, 1 out]
                              }
                              frame "10" {
                                n1377 = local write "midVar_bool_find"(FALSE ("midVar_bool_find")) -> ()
                                n1378 = One Button Dialog(message="工单存在，和料号不匹配！" ("消息")) -> ()  [unwired: 1 in, 1 out]
                              }
                              frame "11" {
                                n1379 = Decimal String To Number(string=w2160) -> (number=w2161:i32)  [unwired: 2 in, 1 out]
                                n1380 = String Subset(string=w2159, length (rest)=5 ("长度（剩余）")) -> (substring=w2157:string)  [unwired: 1 in]
                                n1381 = To Upper Case(1:w2157) -> (0:w2156:string)
                                n1382 = local write "MO Num"(w2161) -> ()
                                n1383 = Equal?(x=w2156, y="E511D") -> (x = y?=w2154:bool)
                                "正常工单?" <- w2154
                                n1384 = case shown="假" w2154 {
                                frame False {
                                n1385 = One Button Dialog(message="不是正常工单号，如测试的是华为料号，\n将不会上传数据到华为，请注意！") -> ()  [unwired: 1 in, 1 out]
                                }
                                frame True {
                                }
                                }
                                n1386 = local write "midVar_bool_find"(TRUE ("midVar_bool_find")) -> ()
                              }
                            }
                          }
                          frame "EE Print" {
                            n1387 = call <vilib>:"Application Directory.vi"() -> ("Application Directory"=w2167:path)
                            n1388 = local read "P/N:"() -> (w2168:string)
                            n1389 = Build Path(base path=w2167, name or relative path="Database\\FigoConfig.xml") -> (appended path=w2165:path)
                            n1390 = call "EEWriteJudge.vi"("path to XML document"=w2165, "PN"=w2168) -> ("Write?"=w2164:bool)  [unwired: 9 in]
                            "EE Write" <- w2164
                            n1391 = local write "midVar_bool_find"(TRUE ("midVar_bool_find")) -> ()
                            n1392 = case shown="假" w2164 {
                              frame False {
                                n1393 = One Button Dialog(message="EE模式不进行烧录") -> ()  [unwired: 1 in, 1 out]
                              }
                              frame True {
                              }
                            }
                          }
                        }
                      }
                      frame #1 {
                        (unwired) "LuxsharePN,CustomerPN,Customer,SampleDes,AWG,Length,EEPROMWrite,LabelPrint,Remarks" ("查询项目")
                        n1394 = call "littleVI_2_part#LabelStr.vi"("input_label"=w2175) -> ("show_label"=→"Label Type":string[])  [unwired: 10 in]
                        n1395 = Index Array(array=w2191, index #1=3 ("索引"), index #2=4 ("索引"), index #3=5 ("索引"), index #4=2 ("索引")) -> (element #1=w2180:string, element #2=w2179:string, element #3=w2178:string, element #4=→"CustomerName":string)
                        "Length" <- w2178
                        n1396 = call "littleVI_1_DesString.vi"("input_Length"=w2178, "input_AWG"=w2179, "input_sampleDes"=w2180) -> ("PNDes"=→"PN Des":string, "SampleDes"=w2177:string)  [unwired: 7 in]
                        n1397 = local write "midVar_bool_find"(TRUE ("midVar_bool_find")) -> ()
                        n1398 = property on="Start Test" class="Bool"("DisabledEnum"=2 ("索引")) -> ()  [unwired: 2 in, 2 out]
                        n1399 = property on="Sample Description" class="Str"("Value"=w2177, "Visible"=TRUE ("可见")) -> ()  [unwired: 2 in, 2 out]
                        n1400 = property on="Result" class="Str"("Visible"=FALSE ("可见"), "Value"="Testing..." ("Result"), "DisabledEnum"=1, "Text.BGColor"=u32 16777216) -> ()  [unwired: 2 in, 2 out]
                        n1401 = local write "labelConfig"(string[] [] ("labelConfig")) -> ()
                      }
                      frame #2 {
                        w2209 = "" ("元素")
                        # "CusPN"
                        # "AWG"
                        n1402 = Index Array(array=w2228, index #1=1 ("索引"), index #2=2 ("索引"), index #3=4 ("索引"), index #4=6 ("索引"), index #8=11 ("索引")) -> (element #1=w2201:string, element #2=→"Cus":string, element #3=w2210:string, element #4=w2226:string, element #5=w2222:string, element #6=w2219:string, element #7=w2216:string, element #8=w2198:string, element #9=w2197:string)  [unwired: 4 in]
                        n1403 = local read "P/N:"() -> (w2213:string)
                        n1404 = call <vilib>:"Trim Whitespace.vi"("string"=w2226) -> ("trimmed string"=w2225:string)  [unwired: 1 in]
                        n1405 = call <vilib>:"Trim Whitespace.vi"("string"=w2198) -> ("trimmed string"=w2207:string)  [unwired: 1 in]
                        n1406 = call <vilib>:"Trim Whitespace.vi"("string"=w2219) -> ("trimmed string"=w2218:string)  [unwired: 1 in]
                        n1407 = call <vilib>:"Trim Whitespace.vi"("string"=w2216) -> ("trimmed string"=w2215:string)  [unwired: 1 in]
                        n1408 = Spreadsheet String To Array(delimiter (Tab)="," ("分隔符(Tab)"), format string="" ("格式字符串"), spreadsheet string=w2197, array type (2D Dbl)=string[] []) -> (array=w2202:string[])
                        n1409 = call <vilib>:"Trim Whitespace.vi"("string"=w2222) -> ("trimmed string"=→"FixtureNo":string)  [unwired: 1 in]
                        n1410 = Equal?(x=w2207, y="1") -> (x = y?=w2196:bool)
                        "AutoSN" <- w2196
                        n1411 = Equal?(x=w2225, y="1") -> (x = y?=→"EEPROMTF":bool)
                        n1412 = Equal?(x=w2218, y="1") -> (x = y?=→"LabelTF":bool)
                        n1413 = Decimal String To Number(string=w2215) -> (number=→"LabelNum":i32)  [unwired: 2 in, 1 out]
                        n1414 = Build Array(w2213, w2210, w2209, w2209, w2201) -> (w2192:string[])
                        "Data In" <- w2192
                        n1415 = local write "frePoints"(w2202) -> ()
                        n1416 = Index Array(array=w2192, index=4 ("索引")) -> (element=w2193:string)
                        n1417 = call <vilib>:"Trim Whitespace.vi"("string"=w2193) -> ("trimmed string"=→"customerPN":string)  [unwired: 1 in]
                        n1418 = case shown="真" w2196 {
                          frame False {
                            n1419 = local write "S/N:"("" ("S/N:")) -> ()
                            n1420 = property on="S/N:" class="Str"("DisabledEnum"=T17."Enabled" ("禁用")) -> ()  [unwired: 2 in, 2 out]
                          }
                          frame True {
                            n1421 = local write "S/N:"("automatic sn" ("S/N:")) -> ()
                            n1422 = property on="S/N:" class="Str"("DisabledEnum"=T17."Disabled and Grayed Out" ("禁用")) -> ()  [unwired: 2 in, 2 out]
                          }
                        }
                      }
                      frame #3 {
                        n1423 = local read "Local Database"() -> (w2233:bool)
                        n1424 = case shown="真" w2233 {
                          tunnel: w2234 -> [_ _]
                          frame False {
                          }
                          frame True {
                          }
                        }
                      }
                      frame #4 {
                        (unwired) FALSE
                        n1425 = local read "EEPROMTF"() -> (w2238:bool)
                        n1426 = local read "Local Database"() -> (w2236:bool)
                        n1427 = case shown="真" w2238 {
                          tunnel: w2237 -> [_ w2240]
                          tunnel: w2236 -> [_ w2239]
                          frame False {
                          }
                          frame True {
                            n1428 = case shown="假" w2239 {
                              tunnel: w2240 -> [_ w2269]
                              frame False {
                                # "此处的mid_array_eep是已经拓展OK的"
                                n1429 = local read "DB2"() -> (w2242:T8)
                                n1430 = local read "DB1"() -> (w2243:T8)
                                n1431 = local read "P/N:"() -> (w2257:string)
                                n1432 = call "getDataFromSQL.vi"("DB"=w2243, "input_str_PN"=w2257) -> ("DateCode8Format_0X30"=w2245:string, "show_str_labelType"=w2252:string, "show_array_eep"=w2254:string[][], "show_bool_valid"=w2255:bool, "show_bool_exsit"=w2256:bool, "show_str_message"=w2253:string, "PN description"=→"PN description":string)  [unwired: 1 out]
                                n1433 = call "boolsToString.vi"("input_bool_low"=w2255, "input_bool_high"=w2256) -> ("show_str_01string"=w2258:string)
                                n1434 = local write "mid_str_labelType"(w2252) -> ()